vi "setup.vi"(3 "Light enables":bool[](array[boolean]), 4 "Calibration file name":path=path "C:/Documents and Settings/ram/My Documents/work/asap/labview/calibration.dat", 5 "Updates/sec":dbl=10.0) -> (0 "error out":errorcluster, 1 "Configuration":T2)   [LabVIEW 2012]
uses:
  configuration.ctl
  asap_calibration.ctl
  <vilib>/Analysis/Matrix/Datatypes/RealMatrix.ctl
  geometry/lut4d.ctl
  globals.vi
  <vilib>/Analysis/Matrix/NI_Matrix.lvlib
panel:
  out "LUT":T1={"Table"=array41x41x41x5x4[1378420 elements], "Scale"=[2.0, 2.0, 2.0, 0.11], "Offset"=[-1.0, -1.0, -1.0, -0.03]}
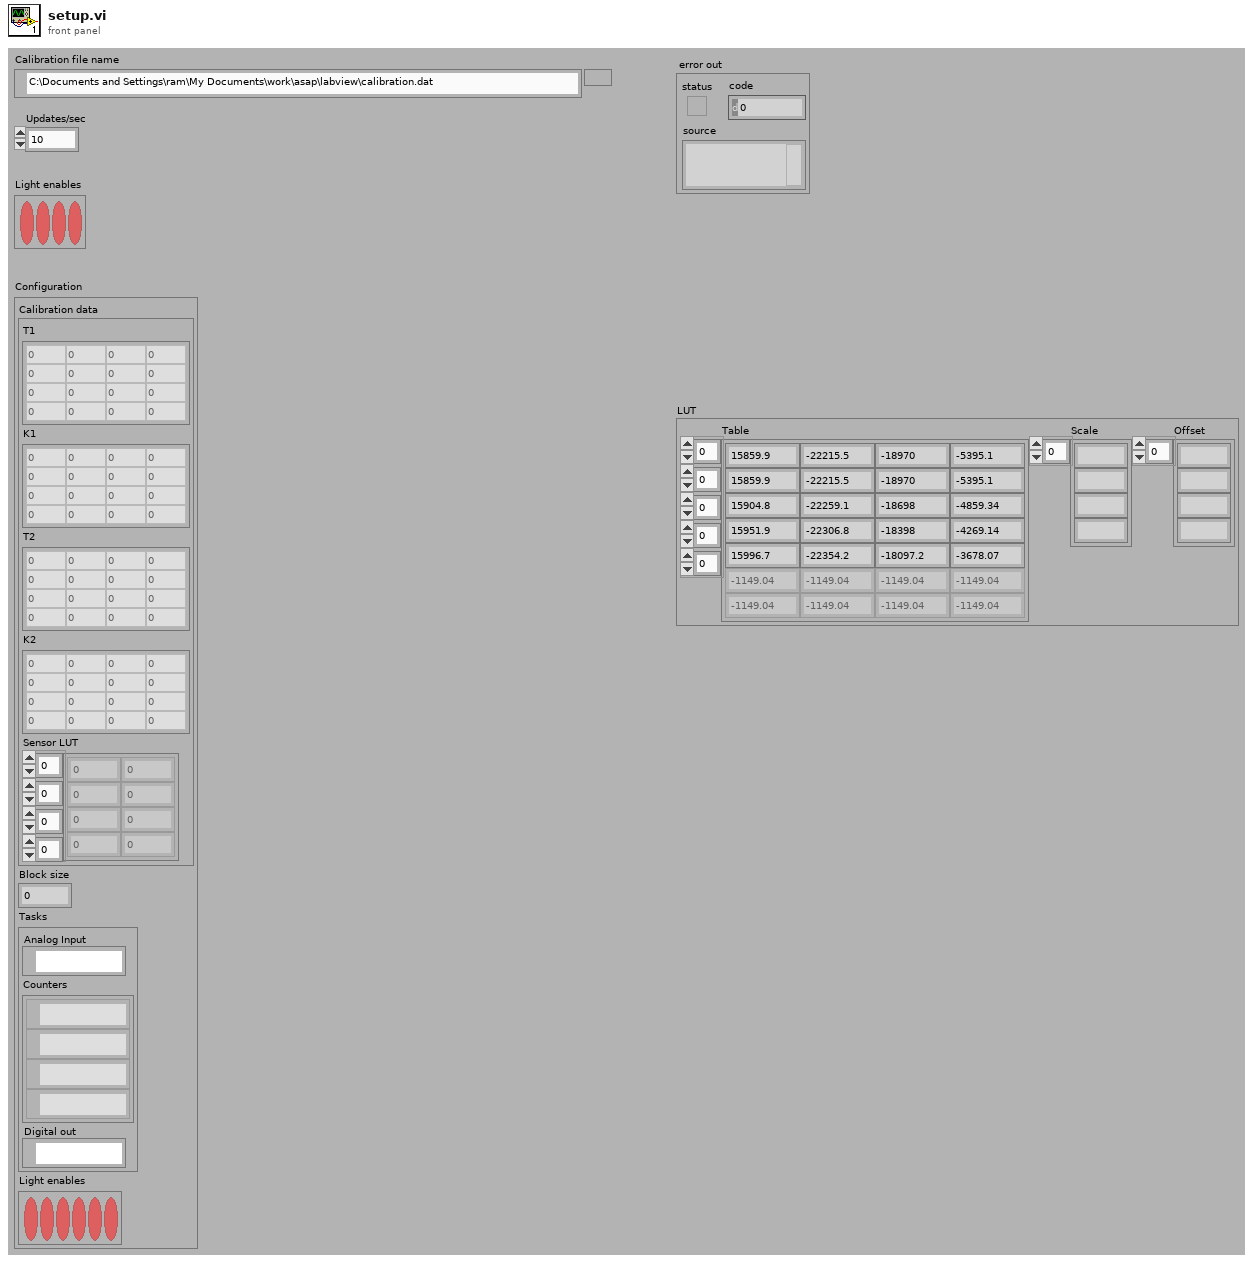
[diagram p1: front panel]
types:
  T1 = typedef "lut4d.ctl" = cluster{"Table":sgl[][][][][], "Scale":sgl[], "Offset":sgl[]}
  T2 = typedef "configuration.ctl" = cluster{"Calibration data":T3, "Block size":i32, "Tasks":cluster{"Analog Input":refnum<k21>, "Counters":refnum<k21>[], "Digital out":refnum<k21>}, "Light enables":bool[]}
  T3 = typedef "asap_calibration.ctl" = cluster{"T1":T4, "K1":T4, "T2":T4, "K2":T4, "Sensor LUT":sgl[][][][]}
  T4 = typedef "NI_Matrix.lvlib/RealMatrix.ctl" = dbl[][]
  T5 = cluster{"Analog Input":refnum<k21>, "Counters":refnum<k21>[], "Digital out":refnum<k21>}
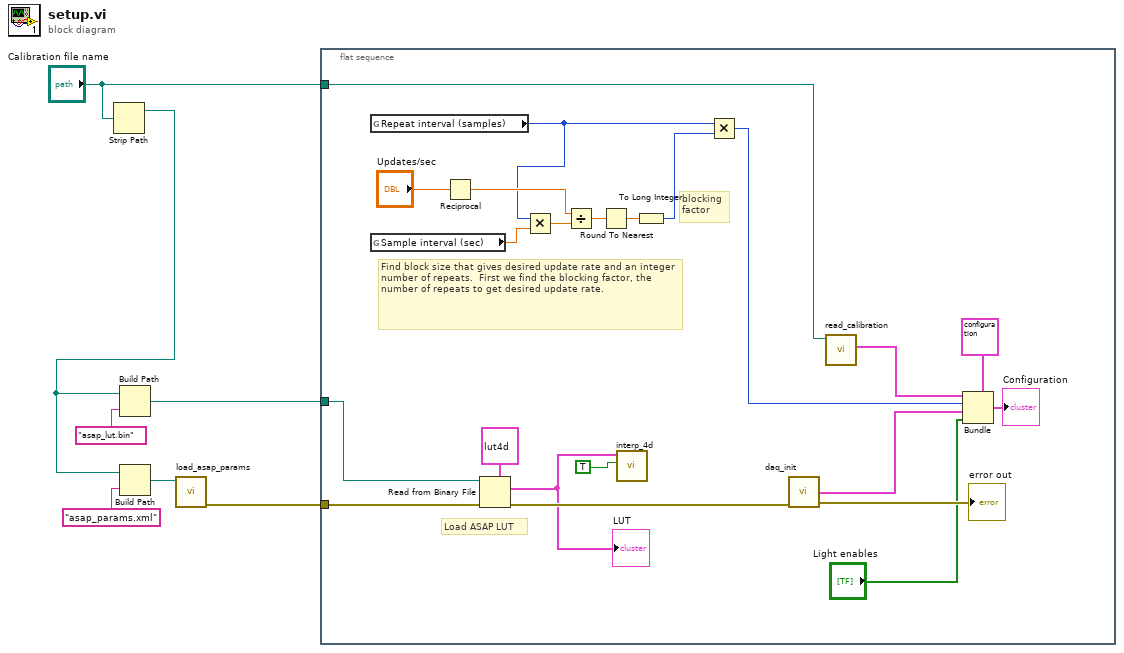
[diagram p0: block diagram]
diagram:
  n1 = Strip Path(path="Calibration file name") -> (stripped path=w2:path)  [unwired: 1 out]
  n2 = Build Path(base path=w2, name or relative path="asap_lut.bin") -> (appended path=w1:path)
  n3 = Build Path(base path=w2, name or relative path="asap_params.xml") -> (appended path=w5:path)
  n4 = call "load_asap_params.vi"("ASAP params file"=w5) -> ("error out"=w4:errorcluster)  [unwired: 1 in, 9 out]
  n5 = flat-sequence {
    tunnel: "Calibration file name" -> [w17]
    tunnel: w4 -> [w14]
    tunnel: w1 -> [w13]
    frame #0 {
      # "Load ASAP LUT"
      # "blocking\nfactor"
      # "Find block size that gives desired update rate and an integer number of repeats.  First we find the blocking factor, the number of repeats to get desired update rate."
      n6 = global read "globals.vi" "Repeat interval (samples)"() -> (w20:i32)
      n7 = global read "globals.vi" "Sample interval (sec)"() -> (w27:dbl)
      n8 = Reciprocal(x="Updates/sec") -> (1/x=w25:dbl)
      n9 = Read from Binary File(5:T1 {"Table"=array41x41x41x5x4[1378420 elements], "Scale"=[2.0, 2.0, 2.0, 0.11], "Offset"=[-1.0, -1.0, -1.0, -0.03]} ("LUT"), 8:w14, 11:w13) -> (0:w15:errorcluster, 2:w12:T1)  [unwired: 5 out]
      "LUT" <- w12
      n10 = Multiply(x=w20, y=w27) -> (x*y=w26:dbl)
      n11 = Divide(x=w25, y=w26) -> (x/y=w23:dbl)
      n12 = Round To Nearest(number=w23) -> (nearest integer value=w22:dbl)
      n13 = call "interp_4d.vi"("Set LUT"=TRUE, "LUT"=w12) -> ()  [unwired: 1 in, 9 out]
      n14 = To Long Integer(number=w22) -> (32bit integer=w21:i32)
      n15 = Multiply(x=w20, y=w21) -> (x*y=w28:i32)
      n16 = call "daq_init.vi"("error in"=w15) -> ("error out"=→"error out":errorcluster, "Tasks"=w19:T5)  [unwired: 4 out]
      n17 = call "read_calibration.vi"("Calibration file name"=w17) -> ("Calibration data"=w29:T3)  [unwired: 1 in, 9 out]
      n18 = Bundle(cluster=T2 {"Calibration data"={"T1"=[], "K1"=[], "T2"=[], "K2"=[], "Sensor LUT"=[]}, "Block size"=0, "Tasks"={"Analog Input"="", "Counters"=[], "Digital out"=""}, "Light enables"=[]} ("Configuration"), "Calibration data"=w29, "Block size"=w28, "Tasks"=w19, "Light enables"="Light enables") -> (→"Configuration":T2)
    }
  }
